vi "UHR-Fleezers Control (host) - 10.8MV_trial.vi"() -> ()   [LabVIEW 2010] (continued)
    n1525 = Multiply(x=10.0, y=w5371) -> (x*y=→"Trap 1 Position RMS (A)":dbl)
    n1526 = Divide(x=w5471, y=w5467) -> (x/y=w5439:waveform(dbl)[])
    n1527 = Index Array(array=w5439, index=0) -> (element=w5449:waveform(dbl))
    n1528 = case "For computing FFTs for display" shown="True" "Compute FFT" {
      tunnel: w5466 -> [_ w7792]
      frame False {
      }
      frame True {
        n1529 = Build Array("FFT 1 Choice 1", "FFT 1 Choice 2", "FFT 2 Choice 1", "FFT 2 Choice 2") -> (w7785:u16[])
        n1530 = Array Size(array=w7792) -> (size(s)=w7791:i32)
        n1531 = feedback-in #6(w7785) -> ()
        n1532 = feedback #6(u16[] [100, 100, 100, 100]) -> (w7786:u16[])
        n1533 = feedback-in #7("# Spectra to Ave.") -> ()
        n1534 = feedback #7("# Spectra to Ave.") -> (w7783:dbl)
        n1535 = Not Equal?(x="# Spectra to Ave.", y=w7783) -> (x != y?=w7782:bool)
        n1536 = Not Equal?(x=w7785, y=w7786) -> (x != y?=w7784:bool)
        n1537 = feedback #8(1.0) -> (w7769:dbl)
        n1538 = Compound Arithmetic op=OR("Reset FFT", w7784, w7782) -> (w7767:bool)
        n1539 = Select(t=1.0, s=w7767, f=w7769) -> (s? t:f=w7771:dbl)
        n1540 = Greater?(x=w7771, y="# Spectra to Ave.") -> (0:w7790:bool)
        n1541 = Increment(x=w7771) -> (x+1=w7770:dbl)
        n1542 = feedback-in #8(w7770) -> ()
        n1543 = local read "DMA Update Period (s)"() -> (w7765:dbl)
        n1544 = Multiply(x="# Spectra to Ave.", y=w7765) -> (x*y=→"Ave. Time (s)":dbl)
        n1545 = Build Array(cluster{"f0":dbl, "df":dbl, "magnitude":dbl[]} {"f0"=0.0, "df"=0.0, "magnitude"=[]} ("PSD")) -> (w7774:cluster{"f0":dbl, "df":dbl, "magnitude":dbl[]}[])
        n1546 = Build Array(w7774, w7774, w7774, w7774) -> (w7776:T49)
        n1547 = feedback #9(w7776) -> (w7781:T49)
        n1548 = for {
          N: 4 -> [_]
          tunnel: w7785 -> [w7814] mode=indexing
          tunnel: w7792 -> [w7815]
          tunnel: w7791 -> [w7817]
          tunnel: w7767 -> [w7810]
          tunnel: w7790 -> [w7809]
          tunnel: "# Spectra to Ave." -> [w7808]
          tunnel: [w7807] -> w7780 mode=indexing
          tunnel: w7781 -> [w7812] mode=indexing
          tunnel: [w7811] -> w7768 mode=indexing
          tunnel: w7771 -> [w7806]
          n1549 = Less?(x=w7814, y=w7817) -> (x < y?=w7816:bool)
          n1550 = Index Array(array=w7815, index=w7814) -> (element=w7813:waveform(dbl))
          n1551 = case shown="True" w7816 {
            tunnel: w7813 -> [_ w7834]
            tunnel: w7812 -> [w7819 w7832]
            tunnel: [w7819 w7820] -> w7811
            tunnel: w7810 -> [_ w7831]
            tunnel: w7809 -> [_ w7824]
            tunnel: w7808 -> [_ w7823]
            tunnel: [cluster{"f0":dbl, "df":dbl, "magnitude":dbl[]} {"f0"=0.0, "df"=0.0, "magnitude"=[]} ("PSD") w7825] -> w7807
            tunnel: w7806 -> [_ w7822]
            frame False {
            }
            frame True {
              n1552 = call <vilib>:"Std Deviation and Variance.vi"("X"=w7834) -> ("mean"=w7835:dbl)  [unwired: 1 in, 2 out]
              n1553 = Subtract(x=w7834, y=w7835) -> (x-y=w7833:waveform(dbl))
              n1554 = xnode "Spectral Measurements"("Signals"=w7833) -> ("PSD"=w7827:cluster{"f0":dbl, "df":dbl, "magnitude":dbl[]})  [unwired: 1 in, 1 out]
              n1555 = case shown="False" w7831 {
                tunnel: w7832 -> [w7844 _]
                tunnel: [w7840 w7849] -> w7820
                tunnel: w7827 -> [w7843 w7850]
                tunnel: w7824 -> [w7842 _]
                frame False {
                  n1556 = Build Array (concatenate)(w7844, w7843) -> (w7841:cluster{"f0":dbl, "df":dbl, "magnitude":dbl[]}[])
                  n1557 = case shown="True" w7842 {
                    tunnel: w7841 -> [w7845 w7848]
                    tunnel: [w7845 w7846] -> w7840
                    frame False {
                    }
                    frame True {
                      n1558 = Delete From Array(array=w7848, index=0) -> (array with subset deleted=w7846:cluster{"f0":dbl, "df":dbl, "magnitude":dbl[]}[])  [unwired: 1 in, 1 out]
                    }
                  }
                }
                frame True {
                  n1559 = Build Array(w7850) -> (w7849:cluster{"f0":dbl, "df":dbl, "magnitude":dbl[]}[])
                }
              }
              n1560 = for {
                tunnel: w7820 -> [w7839] mode=indexing
                tunnel: [w7838] -> w7830 mode=indexing
                workers-P: _ -> [_]
                n1561 = Unbundle By Name(w7839) -> ("magnitude"=w7838:dbl[])
              }
              n1562 = Transpose 2D Array(2D array=w7830) -> (transposed array=w7829:dbl[][])
              n1563 = for {
                tunnel: w7829 -> [w7837] mode=indexing
                tunnel: [w7836] -> w7828 mode=indexing
                workers-P: _ -> [_]
                n1564 = Add Array Elements(numeric array=w7837) -> (sum=w7836:dbl)
              }
              n1565 = Select(t=w7823, s=w7824, f=w7822) -> (s? t:f=w7821:dbl)
              n1566 = Divide(x=w7828, y=w7821) -> (x/y=w7826:dbl[])
              n1567 = Bundle By Name(cluster=w7827, "magnitude"=w7826) -> (w7825:cluster{"f0":dbl, "df":dbl, "magnitude":dbl[]})
            }
          }
        }
        n1568 = case shown="True" w7767 {
          tunnel: w7768 -> [w7799 w7805]
          tunnel: [w7799 w7800] -> w7766
          frame False {
          }
          frame True {
            n1569 = Array Subset(array=w7805, index (row)=0 ("index"), length (row)=4 ("length"), index (col)=0 ("index"), length (col)=1 ("length")) -> (w7800:T49)
          }
        }
        n1570 = feedback-in #9(w7766) -> ()
        n1571 = Split 1D Array(array=w7780, index=2) -> (first subarray=→"FFT 1":cluster{"f0":dbl, "df":dbl, "magnitude":dbl[]}[], second subarray=→"FFT 2":cluster{"f0":dbl, "df":dbl, "magnitude":dbl[]}[])
      }
    }
    n1572 = Index Array(array=w5439, index=1) -> (element=w5447:waveform(dbl))
    n1573 = case "For displaying the high resolution display (no downsampling)" shown="True" w5512 {
      tunnel: w5466 -> [_ w5974]
      frame False {
      }
      frame True {
        n1574 = Index Array(array=w5974, index="High Res. Display") -> (element=w5975:waveform(dbl))
        n1575 = call <vilib>:"Std Deviation and Variance.vi"("X"=w5975) -> ("mean"=w5982:dbl, "standard deviation"=w5987:dbl)  [unwired: 1 in, 1 out]
        "Mean Intensity" <- w5982
        "Sigma" <- w5987
        n1576 = Subtract(x=w5975, y=w5982) -> (x-y=w5981:waveform(dbl))
        n1577 = Select(t=w5981, s="Subtract mean", f=w5975) -> (s? t:f=→"1 Channel":waveform(dbl))
        n1578 = Divide(x=w5987, y=w5982) -> (x/y=→"Sigma/Mean":dbl)
        n1579 = feedback #10(1) -> (w5976:i32)
        n1580 = Greater Or Equal?(x=w5976, y="Slow mean N ave.") -> (x >= y?=w5989:bool)
        n1581 = Increment(x=w5976) -> (x+1=w5991:i32)
        n1582 = Select(t=1, s=w5989, f=w5991) -> (s? t:f=w5978:i32)
        n1583 = feedback-in #10(w5978) -> ()
        n1584 = feedback #11() -> (w5979:waveform(dbl))  [unwired: 1 out]
        n1585 = case shown="Default" w5976 {
          tunnel: [w5994 w5997] -> w5980
          tunnel: w5979 -> [w5996 _]
          tunnel: w5975 -> [w5995 w5997]
          frame Default {
            n1586 = call-poly <vilib>:"Append Waveforms.vi"("waveform B"=w5995, "waveform A"=w5996) -> ("waveform out"=w5994:waveform(dbl))  [unwired: 1 in, 8 out]
          }
          frame 1 {
          }
        }
        n1587 = feedback-in #11(w5980) -> ()
        n1588 = case shown="True" w5989 {
          tunnel: w5980 -> [_ w5993]
          frame False {
          }
          frame True {
            n1589 = call <vilib>:"Mean.vi"("X"=w5993) -> ("mean"=→"Slow mean":dbl)  [unwired: 1 out]
          }
        }
      }
    }
    n1590 = case "For plotting results of scanning MCL" shown="True" w5589 {
      tunnel: w5588 -> [_ w6505]
      tunnel: w5505 -> [_ w6601]
      tunnel: w5597 -> [_ _]
      tunnel: w5466 -> [_ w6575]
      tunnel: w5441 -> [_ w6506]
      tunnel: w5440 -> [_ w6479]
      frame False {
      }
      frame True {
        w6486 = u32 0 items=["Horizontal", "Vertical", "Central", "1st Diagonal", "2nd Diagonal"] ("Type of Symmetry")
        w6514 = u32 0 items=["Horizontal", "Vertical", "Central", "1st Diagonal", "2nd Diagonal"] ("Type of Symmetry")
        w6517 = u32 0 items=["Horizontal", "Vertical", "Central", "1st Diagonal", "2nd Diagonal"] ("Type of Symmetry")
        w6546 = u32 0 items=["Horizontal", "Vertical", "Central", "1st Diagonal", "2nd Diagonal"] ("Type of Symmetry")
        n1591 = Index Array(array=w6575, index=10) -> (element=w6581:waveform(dbl))
        n1592 = Index Array(array=w6575, index=11) -> (element=w6578:waveform(dbl))
        n1593 = local read "Cycles/step (MCL)"() -> (w6531:u64)
        n1594 = Index Array(array=w6575, index="Channel") -> (element=w6577:waveform(dbl))
        n1595 = Unbundle(w6479) -> ("New Image"=w6478:T2, "New Image"=w6477:T2, "New Image"=w6476:T2, "New Image"=w6475:T2)
        n1596 = Unbundle By Name(w6581) -> ("Y"=w6533:dbl[])
        n1597 = Unbundle By Name(w6578) -> ("Y"=w6535:dbl[])
        n1598 = Unbundle By Name(w6577) -> ("Y"=w6540:dbl[])
        n1599 = call "downsample 1D array - double.vi"("Ave N"=w6531, "Array In"=w6533) -> ("Array Out"=w6532:dbl[])  [unwired: 1 out]
        n1600 = call "downsample 1D array - double.vi"("Ave N"=w6531, "Array In"=w6535) -> ("Array Out"=w6534:dbl[])  [unwired: 1 out]
        n1601 = call "downsample 1D array - double.vi"("Ave N"=w6531, "Array In"=w6540) -> ("Array Out"=w6539:dbl[])  [unwired: 1 out]
        n1602 = feedback #12(w6601) -> (w6602:dbl[])
        n1603 = Build Array (concatenate)(w6602, w6601) -> (w6583:dbl[])
        n1604 = feedback #13(w6506) -> (w6508:dbl[])
        n1605 = Build Array (concatenate)(w6508, w6506) -> (w6507:dbl[])
        n1606 = local read "Scan steps (MCL)"() -> (w6488:u64)
        n1607 = Select(t=w6601, s=w6505, f=w6583) -> (s? t:f=w6587:dbl[])
        n1608 = feedback-in #12(w6587) -> ()
        n1609 = Select(t=w6506, s=w6505, f=w6507) -> (s? t:f=w6489:dbl[])
        n1610 = feedback-in #13(w6489) -> ()
        n1611 = local read "Scan lines (y)"() -> (w6474:u64)
        n1612 = local read "N APD Samp/step"() -> (w6490:dbl)
        n1613 = feedback #14(w6532) -> (w6589:dbl[])
        n1614 = Build Array (concatenate)(w6589, w6532) -> (w6580:dbl[])
        n1615 = feedback #15(w6539) -> (w6599:dbl[])
        n1616 = Build Array (concatenate)(w6599, w6539) -> (w6598:dbl[])
        n1617 = feedback #16(w6534) -> (w6591:dbl[])
        n1618 = Build Array (concatenate)(w6591, w6534) -> (w6592:dbl[])
        n1619 = Select(t=w6532, s=w6505, f=w6580) -> (s? t:f=w6536:dbl[])
        n1620 = feedback-in #14(w6536) -> ()
        n1621 = Select(t=w6539, s=w6505, f=w6598) -> (s? t:f=w6538:dbl[])
        n1622 = feedback-in #15(w6538) -> ()
        n1623 = Select(t=w6534, s=w6505, f=w6592) -> (s? t:f=w6537:dbl[])
        n1624 = feedback-in #16(w6537) -> ()
        n1625 = Multiply(x=w6488, y=u64 2) -> (x*y=w6473:u64)
        n1626 = call "integrate 1D array interval - double.vi"("Ave N"=w6490, "Array In"=w6489) -> ("Array Out"=w6501:dbl[])  [unwired: 1 out]
        n1627 = call "integrate 1D array interval - double.vi"("Ave N"=w6490, "Array In"=w6587) -> ("Array Out"=w6586:dbl[])  [unwired: 1 out]
        n1628 = Array Size(array=w6501) -> (size(s)=w6502:i32)
        n1629 = Array Size(array=w6586) -> (size(s)=w6588:i32)
        n1630 = Multiply(x=w6474, y=w6473) -> (x*y=w6504:u64)
        n1631 = Multiply(x=w6474, y=w6473) -> (x*y=w6596:u64)
        n1632 = call <vilib>:"Mean.vi"("X"=w6536) -> ("mean"=w6520:dbl)  [unwired: 1 out]
        n1633 = Subtract(x=w6504, y=w6502) -> (x-y=w6495:u64)
        n1634 = call <vilib>:"Mean.vi"("X"=w6538) -> ("mean"=w6525:dbl)  [unwired: 1 out]
        n1635 = call <vilib>:"Mean.vi"("X"=w6537) -> ("mean"=w6523:dbl)  [unwired: 1 out]
        n1636 = call <vilib>:"Mean.vi"("X"=w6501) -> ("mean"=w6492:dbl)  [unwired: 1 out]
        n1637 = Subtract(x=w6596, y=w6588) -> (x-y=w6530:u64)
        n1638 = call <vilib>:"Mean.vi"("X"=w6586) -> ("mean"=w6527:dbl)  [unwired: 1 out]
        n1639 = Initialize Array(1.0 ("element"), w6495) -> (w6491:dbl[])
        n1640 = Initialize Array(1.0 ("element"), w6530) -> (w6521:dbl[])
        n1641 = Multiply(x=w6491, y=w6492) -> (x*y=w6493:dbl[])
        n1642 = Multiply(x=w6521, y=w6523) -> (x*y=w6524:dbl[])
        n1643 = Multiply(x=w6521, y=w6525) -> (x*y=w6526:dbl[])
        n1644 = Multiply(x=w6521, y=w6520) -> (x*y=w6522:dbl[])
        n1645 = Multiply(x=w6521, y=w6527) -> (x*y=w6528:dbl[])
        n1646 = Build Array (concatenate)(w6536, w6522) -> (w6590:dbl[])
        n1647 = Build Array (concatenate)(w6538, w6526) -> (w6594:dbl[])
        n1648 = Build Array (concatenate)(w6537, w6524) -> (w6593:dbl[])
        n1649 = Build Array (concatenate)(w6501, w6493) -> (w6503:dbl[])
        n1650 = Build Array (concatenate)(w6586, w6528) -> (w6595:dbl[])
        n1651 = Reshape Array(w6590, w6474, w6473) -> (w6556:dbl[][])
        n1652 = Reshape Array(w6503, w6474, w6473) -> (w6499:dbl[][])
        n1653 = Reshape Array(w6594, w6474, w6473) -> (w6548:dbl[][])
        n1654 = Reshape Array(w6593, w6474, w6473) -> (w6563:dbl[][])
        n1655 = Reshape Array(w6595, w6474, w6473) -> (w6573:dbl[][])
        n1656 = Array Subset(array=w6563, index (col)=0 ("index"), length (col)=w6488) -> (w6568:dbl[][])  [unwired: 2 in]
        n1657 = Array Subset(array=w6563, index (col)=w6488) -> (w6566:dbl[][])  [unwired: 3 in]
        n1658 = Array Subset(array=w6548, index (col)=0 ("index"), length (col)=w6488) -> (w6554:dbl[][])  [unwired: 2 in]
        n1659 = Array Subset(array=w6548, index (col)=w6488) -> (w6552:dbl[][])  [unwired: 3 in]
        n1660 = Array Subset(array=w6499, index (col)=0 ("index"), length (col)=w6488) -> (w6498:dbl[][])  [unwired: 2 in]
        n1661 = Array Subset(array=w6499, index (col)=w6488) -> (w6496:dbl[][])  [unwired: 3 in]
        n1662 = Array Subset(array=w6573, index (col)=0 ("index"), length (col)=w6488) -> (w6572:dbl[][])  [unwired: 2 in]
        n1663 = Array Subset(array=w6573, index (col)=w6488) -> (w6570:dbl[][])  [unwired: 3 in]
        n1664 = Array Subset(array=w6556, index (col)=0 ("index"), length (col)=w6488) -> (w6561:dbl[][])  [unwired: 2 in]
        n1665 = Array Subset(array=w6556, index (col)=w6488) -> (w6559:dbl[][])  [unwired: 3 in]
        n1666 = for {
          tunnel: w6568 -> [w6610] mode=indexing
          tunnel: [w6609] -> w6567 mode=indexing
          workers-P: _ -> [_]
          n1667 = Reverse 1D Array(array=w6610) -> (reversed array=w6609:dbl[])
        }
        n1668 = for {
          tunnel: w6554 -> [w6606] mode=indexing
          tunnel: [w6605] -> w6553 mode=indexing
          workers-P: _ -> [_]
          n1669 = Reverse 1D Array(array=w6606) -> (reversed array=w6605:dbl[])
        }
        n1670 = for {
          tunnel: w6498 -> [w6604] mode=indexing
          tunnel: [w6603] -> w6497 mode=indexing
          workers-P: _ -> [_]
          n1671 = Reverse 1D Array(array=w6604) -> (reversed array=w6603:dbl[])
        }
        n1672 = for {
          tunnel: w6572 -> [w6612] mode=indexing
          tunnel: [w6611] -> w6571 mode=indexing
          workers-P: _ -> [_]
          n1673 = Reverse 1D Array(array=w6612) -> (reversed array=w6611:dbl[])
        }
        n1674 = for {
          tunnel: w6561 -> [w6608] mode=indexing
          tunnel: [w6607] -> w6560 mode=indexing
          workers-P: _ -> [_]
          n1675 = Reverse 1D Array(array=w6608) -> (reversed array=w6607:dbl[])
        }
        n1676 = Index Array(array=w6573, index (row)=0) -> (element=→"Waveform Graph":dbl[])  [unwired: 1 in]
        n1677 = Add(x=w6567, y=w6566) -> (x+y=w6565:dbl[][])
        n1678 = Add(x=w6553, y=w6552) -> (x+y=w6551:dbl[][])
        n1679 = Add(x=w6497, y=w6496) -> (x+y=w6481:dbl[][])
        n1680 = Add(x=w6571, y=w6570) -> (x+y=w6545:dbl[][])
        n1681 = Add(x=w6560, y=w6559) -> (x+y=w6558:dbl[][])
        n1682 = Divide(x=w6551, y=2) -> (x/y=w6549:dbl[][])
        n1683 = Divide(x=w6565, y=2) -> (x/y=w6510:dbl[][])
        n1684 = Divide(x=w6558, y=2) -> (x/y=w6512:dbl[][])
        n1685 = To Single Precision Float(number=w6545) -> (single precision float=w6544:sgl[][])
        n1686 = Transpose 2D Array(2D array=w6549) -> (transposed array=→"Data map":dbl[][])
        n1687 = To Single Precision Float(number=w6481) -> (single precision float=w6485:sgl[][])
        n1688 = To Single Precision Float(number=w6510) -> (single precision float=w6516:sgl[][])
        n1689 = To Single Precision Float(number=w6512) -> (single precision float=w6513:sgl[][])
        n1690 = call "IMAQ ArrayToImage"("Image Pixels (Float)"=w6544, "Image"=w6478) -> ("Image Out"=w6547:T2)  [unwired: 8 in, 1 out]
        n1691 = call "IMAQ ArrayToImage"("Image Pixels (Float)"=w6485, "Image"=w6477) -> ("Image Out"=w6487:T2)  [unwired: 8 in, 1 out]
        n1692 = call "IMAQ ArrayToImage"("Image Pixels (Float)"=w6516, "Image"=w6476) -> ("Image Out"=w6518:T2)  [unwired: 8 in, 1 out]
        n1693 = call "IMAQ ArrayToImage"("Image Pixels (Float)"=w6513, "Image"=w6475) -> ("Image Out"=w6515:T2)  [unwired: 8 in, 1 out]
        n1694 = call "IMAQ Symmetry"("Type of Symmetry"=w6546, "Image Src"=w6547) -> ("Image Dst Out"=w6542:T2)  [unwired: 3 in, 1 out]
        n1695 = call "IMAQ Symmetry"("Type of Symmetry"=w6486, "Image Src"=w6487) -> ("Image Dst Out"=w6483:T2)  [unwired: 3 in, 1 out]
        n1696 = call "IMAQ Symmetry"("Type of Symmetry"=w6517, "Image Src"=w6518) -> ("Image Dst Out"=→"Detection Laser X":T2)  [unwired: 3 in, 1 out]
        n1697 = call "IMAQ Symmetry"("Type of Symmetry"=w6514, "Image Src"=w6515) -> ("Image Dst Out"=→"Detection Laser Y":T2)  [unwired: 3 in, 1 out]
        n1698 = call "IMAQ Set Simple Calibration"("Calibration Axis Info"=T38 {"Origin Pixel"={"X"=0.0, "Y"=0.0}, "Angle Relative to Horizontal (deg)"=0.0, "Axis Reference"=0}, "Grid Descriptor"=T39 {"X Step"=0.3, "Y Step"=0.3, "Unit"=enum."Undefined"}, "Image"=w6542) -> ("Calibrated Image"=→"APD 1":T2)  [unwired: 7 in, 1 out]
        n1699 = call "IMAQ Set Simple Calibration"("Calibration Axis Info"=T38 {"Origin Pixel"={"X"=0.0, "Y"=0.0}, "Angle Relative to Horizontal (deg)"=0.0, "Axis Reference"=0}, "Grid Descriptor"=T39 {"X Step"=0.3, "Y Step"=0.3, "Unit"=enum."Undefined"}, "Image"=w6483) -> ("Calibrated Image"=→"APD 2":T2)  [unwired: 7 in, 1 out]
      }
    }
    n1700 = Subtract(x=w5447, y="APD 2 Offset") -> (x-y=w5444:waveform(dbl))
    n1701 = Subtract(x=w5449, y="APD 1 Offset") -> (x-y=w5445:waveform(dbl))
    n1702 = Index Array(array=w5464, index=3) -> (element=w5533:waveform(dbl))
    n1703 = Index Array(array=w5464, index=6) -> (element=w5530:waveform(dbl))
    n1704 = Build Array(w5445, w5444) -> (→"APD Chart":waveform(dbl)[])
    n1705 = Array Size(array=w5522) -> (size(s)=w5577:i32)
    n1706 = call <vilib>:"Std Deviation and Variance.vi"("X"=w5457) -> ("standard deviation"=w5456:dbl)  [unwired: 1 in, 2 out]
    n1707 = Add Array Elements(numeric array=w5457) -> (sum=w5459:u32)
    n1708 = Add Array Elements(numeric array=w5522) -> (sum=w5587:u32)
    n1709 = call <vilib>:"Std Deviation and Variance.vi"("X"=w5522) -> ("standard deviation"=w5521:dbl)  [unwired: 1 in, 2 out]
    n1710 = Divide(x="T1 offset_x (mV)", y=1000.0) -> (x/y=w5534:dbl)
    n1711 = Divide(x=w5456, y=w5455) -> (x/y=w5452:dbl)
    "Rate sigma (Hz) 2" <- w5452
    n1712 = Multiply(x=w5455, y=w5577) -> (x*y=w5458:dbl)
    "Int. Time (s)" <- w5458
    n1713 = Divide(x=w5459, y=w5458) -> (x/y=w5453:dbl)
    "APD 2 Rate (Hz)" <- w5453
    n1714 = Divide(x=w5587, y=w5458) -> (x/y=w5519:dbl)
    "APD 1 Rate (Hz)" <- w5519
    n1715 = Divide(x=w5521, y=w5455) -> (x/y=w5520:dbl)
    "Rate sigma (Hz)" <- w5520
    n1716 = Divide(x=w5452, y=w5453) -> (x/y=→"Sigma/Mean 2":dbl)
    n1717 = Divide(x=w5520, y=w5519) -> (x/y=→"Sigma/Mean":dbl)
    n1718 = Divide(x="T2 offset_x (mV)", y=1000.0) -> (x/y=w5532:dbl)
    n1719 = case shown="1" "Calibration" {
      tunnel: "T1 alpha_x (nm/V)" -> [_ w6441 w6462]
      tunnel: "T1 kappa_x (pN/nm)" -> [_ _ w6452]
      tunnel: "T2 alpha_x (nm/V)" -> [_ w6440 w6460]
      tunnel: "T2 kappa_x (pN/nm)" -> [_ _ w6453]
      tunnel: w5533 -> [w6423 w6438 w6458]
      tunnel: w5530 -> [w6422 w6436 w6456]
      tunnel: [w6423 w6435 w6455] -> w5563
      tunnel: [w6422 w6434 w6454] -> w5562
      tunnel: ["T1 X (V)" ("Label.Text") "T1 X (nm)" ("Label.Text") "T1 X (pN)" ("Label.Text")] -> w5551
      tunnel: ["T2 X (V)" ("Label.Text") "T2 X (nm)" ("Label.Text") "T2 X (pN)" ("Label.Text")] -> w5550
      tunnel: ["Position (V)" ("Label.Text") "Position (nm)" ("Label.Text") "Force (pN)" ("Label.Text")] -> w5552
      tunnel: w5532 -> [_ w6426 w6445]
      tunnel: w5534 -> [_ w6429 w6447]
      tunnel: ["Mean (V)" ("Label.Text") "Mean (nm)" ("Label.Text") "Mean (pN)" ("Label.Text")] -> w5547
      tunnel: ["Difference (V)" ("Label.Text") "Difference (nm)" ("Label.Text") "Difference (pN)" ("Label.Text")] -> w5472
      frame 0, Default {
      }
      frame 1 {
        # "position"
        n1720 = Unbundle By Name(w6438) -> ("Y"=w6442:dbl[])
        n1721 = Unbundle By Name(w6436) -> ("Y"=w6427:dbl[])
        n1722 = Subtract(x=w6442, y=w6429) -> (x-y=w6430:dbl[])
        n1723 = Subtract(x=w6427, y=w6426) -> (x-y=w6428:dbl[])
        n1724 = Multiply(x=w6428, y=w6440) -> (x*y=w6437:dbl[])
        n1725 = Multiply(x=w6441, y=w6430) -> (x*y=w6439:dbl[])
        n1726 = Bundle By Name(cluster=w6436, "Y"=w6437) -> (w6434:waveform(dbl))
        n1727 = Bundle By Name(cluster=w6438, "Y"=w6439) -> (w6435:waveform(dbl))
      }
      frame 2 {
        # "force"
        n1728 = Unbundle By Name(w6458) -> ("Y"=w6463:dbl[])
        n1729 = Unbundle By Name(w6456) -> ("Y"=w6461:dbl[])
        n1730 = Subtract(x=w6461, y=w6445) -> (x-y=w6446:dbl[])
        n1731 = Subtract(x=w6463, y=w6447) -> (x-y=w6448:dbl[])
        n1732 = Compound Arithmetic op=MULTIPLY(w6446, w6460, w6453) -> (w6457:dbl[])
        n1733 = Compound Arithmetic op=MULTIPLY(w6452, w6462, w6448) -> (w6459:dbl[])
        n1734 = Bundle By Name(cluster=w6456, "Y"=w6457) -> (w6454:waveform(dbl))
        n1735 = Bundle By Name(cluster=w6458, "Y"=w6459) -> (w6455:waveform(dbl))
      }
    }
    n1736 = feedback-in #17("Calibration") -> ()
    n1737 = feedback #17(u16 1 ("Calibration")) -> (w5554:u16)
    n1738 = Not Equal?(x=w5554, y="Calibration") -> (x != y?=w5510:bool)
    n1739 = Unbundle By Name(w5533) -> ("Y"=w5536:dbl[])
    n1740 = Unbundle By Name(w5530) -> ("Y"=w5539:dbl[])
    n1741 = Subtract(x=w5536, y=w5534) -> (x-y=w5537:dbl[])
    n1742 = Subtract(x=w5539, y=w5532) -> (x-y=w5538:dbl[])
    n1743 = disable-structure shown="Enabled" {
      disable-tunnel: [-1.0 ("y") 1.0] -> w5540
      frame Disabled {
      }
      frame Enabled {
      }
    }
    n1744 = Multiply(x=w5538, y="T2 alpha_x (nm/V)") -> (x*y=w5529:dbl[])
    n1745 = Multiply(x="T1 alpha_x (nm/V)", y=w5537) -> (x*y=w5528:dbl[])
    n1746 = Multiply(x=w5562, y=w5540) -> (x*y=w5541:waveform(dbl))
    n1747 = case shown="True" "Read Lateness and Rel Phase" {
      tunnel: w5364 -> [w5998 w6020]
      tunnel: w5363 -> [w5999 w6019]
      tunnel: [w5998 w6018] -> w5525
      tunnel: [w5999 w6017] -> w5524
      frame False {
      }
      frame True {
        n1748 = xnode "Read/Write Control"("FPGA VI Reference In"=w6020, "error in"=w6019) -> ("FPGA VI Reference Out"=w6018:T19, "error out"=w6017:errorcluster, "GI Relative phase"=→"GI relative phase":i16, "Relative phase"=→"Relative phase (AI1)":i16, "AI Late Counter"=→"Late Counter (AI1)":u16, "GI Late Counter"=→"GI Late Counter":u16, "MCL Late Counter"=→"MCL Late Counter":u16, "MCL Relative Phase"=→"Relative Phase (MCL)":i16, "APD Acq Relative Phase"=→"APD Acq Relative Phase":i16, "APD 1 Gate Relative Phase"=→"APD 1 Gate Relative Phase":i16, "APD 2 Gate Relative Phase"=→"APD 2 Gate Relative Phase":i16, "APD Acq Late Counter"=→"APD Acq Late Counter":u16, "APD 1 Gate Late Counter"=→"APD 1 Gate Late Counter":u16, "APD 2 Gate Late Counter"=→"APD 2 Gate Late Counter":u16, "Green FB Relative Phase"=→"Relative phase (Green FB)":i16, "GI Relative phase 2"=→"GI relative phase 2":i16, "GI Late Counter 2"=→"GI Late Counter 2":u16, "Trap Pos FIFO Timeout"=→"Trap Pos FIFO Timeout":u16, "Trap AI FIFO Timeout"=→"Trap AI FIFO Timeout":u16)
      }
    }
    n1749 = Subtract(x=w5529, y=w5528) -> (x-y=w5527:dbl[])
    n1750 = Unbundle By Name(w5562) -> ("Y"=w5497:dbl[])
    n1751 = Unbundle By Name(w5563) -> ("Y"=w5498:dbl[])
    n1752 = Build Array(w5563, w5541) -> (→"Force":waveform(dbl)[])
    n1753 = Subtract(x=w5527, y="Offset (nm)") -> (x-y=w5495:dbl[])
    n1754 = call <vilib>:"Mean.vi"("X"=w5497) -> ("mean"=w5476:dbl)  [unwired: 1 out]
    "T2 X" <- w5476
    n1755 = Absolute Value(x=w5498) -> (abs(x)=w5499:dbl[])
    n1756 = Absolute Value(x=w5497) -> (abs(x)=w5500:dbl[])
    n1757 = call <vilib>:"Mean.vi"("X"=w5498) -> ("mean"=w5477:dbl)  [unwired: 1 out]
    "T1 X" <- w5477
    n1758 = Add(x=w5499, y=w5500) -> (x+y=w5501:dbl[])
    n1759 = Bundle By Name(cluster=w5533, "Y"=w5495) -> (w5463:waveform(dbl))
    "Bead Separation" <- w5463
    n1760 = Divide(x=w5501, y=2.0) -> (x/y=→"Vec Mean of T1 T2":dbl[])
    n1761 = case shown="True" w5510 {
      tunnel: w5552 -> [_ w6416]
      tunnel: w5551 -> [_ w6415]
      tunnel: w5550 -> [_ w6414]
      tunnel: w5547 -> [_ w6413]
      tunnel: w5472 -> [_ w6412]
      frame False {
      }
      frame True {
        n1762 = property on="Force" class="WFChart (strict)"("YScale.NameLbl.Text"=w6416) -> ()  [unwired: 2 in, 2 out]
        n1763 = property on="T2 X" class="DigNum (strict)"("Caption.Text"=w6414) -> ()  [unwired: 2 in, 2 out]
        n1764 = property on="T1 X" class="DigNum (strict)"("Caption.Text"=w6415) -> ()  [unwired: 2 in, 2 out]
        n1765 = property on="Mean" class="DigNum (strict)"("Caption.Text"=w6413) -> ()  [unwired: 2 in, 2 out]
        n1766 = property on="Difference" class="DigNum (strict)"("Caption.Text"=w6412) -> ()  [unwired: 2 in, 2 out]
      }
    }
    n1767 = local read "Tether"() -> (w5504:bool)
    n1768 = Absolute Value(x=w5477) -> (abs(x)=w5474:dbl)
    n1769 = Absolute Value(x=w5476) -> (abs(x)=w5473:dbl)
    n1770 = Add(x=w5474, y=w5473) -> (x+y=w5549:dbl)
    n1771 = Subtract(x=w5474, y=w5473) -> (x-y=→"Difference":dbl)
    n1772 = feedback #18(w5495) -> (w5494:dbl[])
    n1773 = Divide(x=w5549, y=2.0) -> (x/y=w5503:dbl)
    "Mean" <- w5503
    n1774 = case shown="True" w5504 {
      tunnel: w5503 -> [_ w5957]
      frame False {
      }
      frame True {
        n1775 = Greater?(x="Lost Tether Alarm Threshold (pN)", y=w5957) -> (0:w5955:bool)
        n1776 = case shown="True" w5955 {
          frame False {
          }
          frame True {
            n1777 = flat-sequence {
              frame #0 {
                # "stop only if saving"
                n1778 = local read "Saving..."() -> (w5970:bool)
                n1779 = And(x=w5970, y="TA Cancel Save?") -> (x .and. y?=w5969:bool)
                n1780 = local write "Stop Saving"(w5969) -> ()
              }
              frame #1 {
                n1781 = case shown="True" "TA Green Off?" {
                  frame False {
                  }
                  frame True {
                    w5973 = FALSE ("Fl. Triggered...")
                    n1782 = local write "Fl. Triggered..."(w5973) -> ()
                    n1783 = property on="Green Laser ON/Interlacing" class="Bool (strict)"("Val(Sgnl)"=w5973) -> ()  [unwired: 2 in, 2 out]
                  }
                }
              }
            }
            n1784 = local read "Time tether formed"() -> (w5964:timestamp)
            n1785 = Get Date/Time In Seconds() -> (seconds since 1Jan1904=w5965:timestamp)
            n1786 = Subtract(x=w5965, y=w5964) -> (x-y=w5963:dbl)
            n1787 = Number To Decimal String(number=w5963) -> (decimal integer string=w5960:string)  [unwired: 1 out]
            n1788 = local read "Messages"() -> (w5967:string)
            n1789 = call <vilib>:"Beep.vi"() -> ()  [unwired: 3 in, 9 out]
            n1790 = Concatenate Strings("Lost tether (" ("Message to add"), w5960, " s)." ("string")) -> (w5962:string)
            n1791 = local write "Tether"(FALSE ("Tether")) -> ()
            n1792 = call "Update messages.vi"("Message to add"=w5962, "Old message string"=w5967) -> ("New message string"=w5966:string)
            n1793 = local write "Messages"(w5966) -> ()
            n1794 = property on="Trap Pos. FB ON" class="Bool (strict)"("Val(Sgnl)"=FALSE ("Value (Signaling)")) -> ()  [unwired: 2 in, 2 out]
          }
        }
      }
    }
    n1795 = Build Array (concatenate)(w5495, w5494) -> (w5493:dbl[])
    n1796 = Split 1D Array(array=w5493, index=w5375) -> (first subarray=w5489:dbl[])  [unwired: 1 out]
    n1797 = feedback-in #18(w5489) -> ()
    n1798 = call <vilib>:"Mean.vi"("X"=w5489) -> ("mean"=w5488:dbl)  [unwired: 1 out]
    "Bead Mean (nm)" <- w5488
    n1799 = Subtract(x=w5489, y=w5488) -> (x-y=w5487:dbl[])
    n1800 = Square(x=w5487) -> (x^2=w5486:dbl[])
    n1801 = call <vilib>:"Mean.vi"("X"=w5486) -> ("mean"=w5485:dbl)  [unwired: 1 out]
    n1802 = Square Root(x=w5485) -> (sqrt(x)=w5484:dbl)
    n1803 = Multiply(x=10.0, y=w5484) -> (x*y=→"RMS (Ang)":dbl)
    n1804 = xnode "Read/Write Control"("FPGA VI Reference In"=w5525, "error in"=w5524) -> ("FPGA VI Reference Out"=w5643:T19, "error out"=w5637:errorcluster, "AI2 Y Sum Set 1"=w5633:i16, "AI2 Y Sum Set 2"=w5632:i16, "AI1 X Set 1"=w5409:fxp<+/-,16,1>, "AI1 X Set 2"=w5408:fxp<+/-,16,1>, "Trap Pos FB Int Signal"=→"Trap Pos FB Int Signal":fxp<+/-,24,9>, "Trap Pos FB Int-Norm Signal"=→"Trap Pos FB Int-Norm Signal":fxp<+/-,16,1>, "Trap Pos FB Action"=w5402:i64, "Scanning"=→"AOD Scanning":bool, "Scan I"=→"AOD Scan I":u64, "Scanning MCL"=w5635:bool, "Scan I (MCL)"=→"MCL Scan I":u64, "Green FB Signals"=w5572:T43)  [unwired: 1 out]
    "MCL Scanning" <- w5635
    "Trap Pos FB Action" <- w5402
    n1805 = local read "AI2 (V)"() -> (w5634:cluster{"Set 1":dbl, "Set 2":dbl})
    n1806 = Bundle By Name(cluster=w5634, "Set 1"=w5633, "Set 2"=w5632) -> (w5630:cluster{"Set 1":dbl, "Set 2":dbl})
    n1807 = Divide(x=w5402, y=327.67) -> (x/y=→"Action (%)":dbl)
    n1808 = local read "Trap X (AI1)"() -> (w5422:T10)
    n1809 = Divide(x=w5630, y=3276.7) -> (x/y=w5629:cluster{"Set 1":dbl, "Set 2":dbl})
    n1810 = local write "AI2 (V)"(w5629) -> ()
    n1811 = Bundle(cluster=w5422, "Trap 1"=w5409, "Trap 2"=w5408) -> (→"Trap X (AI1)":T10)
    n1812 = Divide(x=w5572, y=3276.7) -> (x/y=w5568:T50)
    n1813 = Unbundle By Name(w5568) -> ("Green FB Ch 0"=w5571:dbl, "Green FB Ch 1"=w5570:dbl, "Green FB Ch 2"=w5569:dbl)
    n1814 = Divide(x=w5571, y=w5569) -> (x/y=w5567:dbl)
    n1815 = Divide(x=w5570, y=w5569) -> (x/y=w5566:dbl)
    n1816 = flat-sequence "To save data" {
      tunnel: [w8273] -> w5654
      tunnel: [w8274] -> w5653
      tunnel: w5603 -> [w8267]
      tunnel: w5491 -> [w8271]
      tunnel: ["Save Calibration"] -> w5626
      tunnel: w5623 -> [w8270]
      tunnel: [w8263] -> w5622
      tunnel: [w8260] -> w5621
      tunnel: [w8257] -> w5620
      tunnel: w5602 -> [w8259]
      tunnel: w5508 -> [w8253]
      tunnel: [w8253] -> w5507
      tunnel: ["Start Saving"] -> w5465
      tunnel: [w8247] -> w5391
      tunnel: [w8246] -> w5390
      tunnel: w5654 -> [w8508]
      tunnel: w5653 -> [w8507]
      tunnel: w5392 -> [w8506]
      tunnel: w5626 -> [w8505]
      tunnel: w5622 -> [w8503]
      tunnel: w5621 -> [w8502]
      tunnel: w5620 -> [w8501]
      tunnel: w5478 -> [w8500]
      tunnel: w5517 -> [w8499]
      tunnel: w5507 -> [w8498]
      tunnel: w5465 -> [w8497]
      tunnel: w5463 -> [w8496]
      tunnel: w5439 -> [w8495]
      tunnel: w5391 -> [w8494]
      tunnel: w5390 -> [w8493]
      tunnel: w5389 -> [w8492]
      frame #0 {
        n1817 = Or(x="Save N Sets", y="Start Saving") -> (x .or. y?=w8254:bool)
        n1818 = To Double Precision Float(number=w8270) -> (double precision float=w8264:dbl)
        n1819 = Build Array(w8254, "Save Calibration", w8267, w8259) -> (w8269:bool[])
        n1820 = Compound Arithmetic op=OR("Save Calibration", w8267, w8254, w8259) -> (w8272:bool)
        n1821 = Boolean Array To Number(Boolean array=w8269) -> (number=w8266:u32)
        n1822 = feedback #19(FALSE ("Save APD Data\nwith Trap Data")) -> (w8248:bool)
        n1823 = feedback #20(refnum<k0> refnum) -> (w8275:refnum<file>)
        n1824 = feedback #21(refnum<k0> refnum) -> (w8250:refnum<file>)
        n1825 = feedback #22(FALSE ("Save APD Data\nwith Trap Data")) -> (w8258:bool)
        n1826 = feedback #23(refnum<k0> refnum) -> (w8261:refnum<file>)
        n1827 = feedback #24(0) -> (w8277:i32)
        n1828 = feedback #25() -> (w8265:u32)  [unwired: 1 out]
        n1829 = case shown="True" w8272 {
          tunnel: [w8284 1] -> w8273
          tunnel: w8277 -> [w8286 _]
          tunnel: [w8285 w8304] -> w8274
          tunnel: w8275 -> [w8285 _]
          tunnel: w8271 -> [_ w8324]
          tunnel: w8264 -> [_ w8322]
          tunnel: w8266 -> [_ w8325]
          tunnel: [w8283 w8303] -> w8263
          tunnel: w8265 -> [w8283 _]
          tunnel: [w8282 w8301] -> w8260
          tunnel: w8261 -> [w8282 _]
          tunnel: [w8281 w8300] -> w8257
          tunnel: w8258 -> [w8281 _]
          tunnel: "Start Saving" -> [_ w8298]
          tunnel: w8253 -> [_ w8297]
          tunnel: [w8280 w8288] -> w8246
          tunnel: w8250 -> [w8280 _]
          tunnel: [w8279 w8287] -> w8247
          tunnel: w8248 -> [w8279 _]
          frame False {
            n1830 = Increment(x=w8286) -> (x+1=w8284:i32)
          }
          frame True {
            w8294 = FALSE ("Start Saving")
            w8299 = 9.0  # File Version
            w8307 = FALSE ("prepend array or string size? (T)")
            w8305 = T31."big-endian, network order" ("byte order (0:big-endian, network order)")
            # "write file headers"
            n1831 = local read "BD 1 Frequency 1 (MHz)"() -> (w8321:dbl)
            n1832 = local read "BD 2 Frequency 1 (MHz)"() -> (w8320:dbl)
            n1833 = local read "BD 1 Frequency 2 (MHz)"() -> (w8319:dbl)
            n1834 = local read "BD 2 Frequency 2 (MHz)"() -> (w8318:dbl)
            n1835 = local read "BD 1 Frequency 3 (MHz)"() -> (w8317:dbl)
            n1836 = local read "BD 2 Frequency 3 (MHz)"() -> (w8316:dbl)
            n1837 = Array Size(array=w8297) -> (size(s)=w8296:i32)
            n1838 = To Double Precision Float(number=w8296) -> (double precision float=w8295:dbl)
            n1839 = local write "Save Calibration"(w8294) -> ()
            n1840 = local write "Start Saving"(w8294) -> ()
            n1841 = Build Array("Save APD Data\nwith Trap Data", "Save Trap Pos. Data") -> (w8291:bool[])
            n1842 = Boolean Array To Number(Boolean array=w8291) -> (number=w8290:u32)
            n1843 = Build Array(w8321, w8320, w8319, w8318, w8317, w8316) -> (w8315:dbl[])
            n1844 = case shown="4" w8325 {
              tunnel: w8324 -> [w8396 w8416 w8432 w8470]
              tunnel: w8295 -> [w8401 w8423 w8452 w8489]
              tunnel: w8322 -> [w8400 w8422 w8451 w8488]
              tunnel: [w8397 w8418 w8443 w8480] -> w8313
              tunnel: [w8388 "Cal sets to save" w8433 w8471] -> w8303
              tunnel: w8315 -> [w8398 w8419 w8445 w8482]
              tunnel: "Save APD Data\nwith Trap Data" -> [w8395 _ w8429 w8468]
              tunnel: [w8395 w8410 w8429 w8468] -> w8300
              tunnel: w8299 -> [w8391 w8411 w8427 w8466]
              tunnel: w8298 -> [w8390 _ _ _]
              tunnel: [w8381 w8410 w8426 w8456] -> w8287
              tunnel: "Save Trap Pos. Data" -> [w8381 _ w8426 w8456]
              tunnel: w8290 -> [w8380 _ w8425 w8455]
              frame 1, Default {
                # "timeseries"
                n1845 = case shown="True" "Profile" {
                  tunnel: [w8404 w8407] -> w8385
                  tunnel: [w8404 w8406] -> w8384
                  tunnel: [w8404 w8405] -> w8383
                  tunnel: [w8404 w8409] -> w8382
                  frame False {
                    w8404 = 0.0 ("f")
                  }
                  frame True {
                    n1846 = local read "Current Position"() -> (w8408:dbl[])
                    n1847 = local read "Y change (mm)"() -> (w8409:dbl)
                    n1848 = call "subVI_explode3array.vi"("Array"=w8408) -> ("x"=w8407:dbl, "y"=w8406:dbl, "z"=w8405:dbl)  [unwired: 12 in]
                  }
                }
                n1849 = local read "Save ave N"() -> (w8403:dbl)
                n1850 = Multiply(x=w8403, y=w8396) -> (x*y=w8402:dbl)
                n1851 = To Double Precision Float(number=w8380) -> (double precision float=w8394:dbl)
                n1852 = Build Array(w8391, w8396, w8402, w8401, w8400, 0.0 ("f")) -> (w8399:dbl[])
                n1853 = Build Array(w8394, w8385, w8384, w8383, w8382) -> (w8392:dbl[])
                n1854 = Select(t=u32 4000000000, s=w8390, f="N sets to save") -> (s? t:f=w8388:u32)
                n1855 = Build Array (concatenate)(w8399, w8398, w8392) -> (w8397:dbl[])
              }
              frame 2 {
                w8413 = 0.0 ("f")
                w8410 = FALSE ("Save APD Data\nwith Trap Data")
                # "calibration"
                n1856 = Boolean To (0,1)(Boolean=w8410) -> (0, 1=w8415:i16)
                n1857 = To Double Precision Float(number=w8415) -> (double precision float=w8414:dbl)
                n1858 = Build Array(w8414, w8413, w8413, w8413, w8413) -> (w8412:dbl[])
                n1859 = Build Array(w8411, w8416, w8416, w8423, w8422, 1.0 ("t")) -> (w8420:dbl[])
                n1860 = Build Array (concatenate)(w8420, w8419, w8412) -> (w8418:dbl[])
                "Calibrating Trap..." <- TRUE ("Calibrating...")
              }
              frame 4 {
                w8430 = 0.0 ("f")
                # "write file header for a trap \nraster scan"
                # "scan dir (x/y = 0/1)"
                # "cycles/step"
                # "n scans (f/b)"
                # "steps"
                # "freq. range"
                # "AOD raster scan"
                n1861 = local read "Number of F/B Scans (AOD)"() -> (w8437:u16)
                n1862 = local read "Cycles/step (AOD)"() -> (w8439:u64)
                n1863 = local read "Scan Range (MHz)"() -> (w8442:dbl)
                n1864 = local read "Scan steps (AOD)"() -> (w8441:u64)
                n1865 = local read "Scan BD"() -> (w8449:bool)
                n1866 = local read "Save ave N"() -> (w8454:dbl)
                n1867 = Boolean To (0,1)(Boolean=w8449) -> (0, 1=w8448:i16)
                n1868 = To Double Precision Float(number=w8437) -> (double precision float=w8436:dbl)
                n1869 = To Double Precision Float(number=w8441) -> (double precision float=w8440:dbl)
                n1870 = To Double Precision Float(number=w8439) -> (double precision float=w8438:dbl)
                n1871 = To Double Precision Float(number=w8448) -> (double precision float=w8447:dbl)
                n1872 = Multiply(x=w8454, y=w8432) -> (x*y=w8453:dbl)
                n1873 = To Double Precision Float(number=w8425) -> (double precision float=w8431:dbl)
                n1874 = Build Array(w8431, w8430, w8430, w8430, w8430) -> (w8428:dbl[])
                n1875 = local read "N sets should be saved"() -> (w8434:dbl)
                n1876 = Build Array(w8447, w8442, w8440, w8438, w8436) -> (w8444:dbl[])
                n1877 = Build Array(w8427, w8432, w8453, w8452, w8451, 2.0 ("t")) -> (w8446:dbl[])
                n1878 = Round Toward +Infinity(x=w8434) -> (ceil(x): smallest int >= x=w8435:dbl)
                n1879 = Build Array (concatenate)(w8446, w8445, w8428, w8444) -> (w8443:dbl[])
                n1880 = To Unsigned Long Integer(number=w8435) -> (unsigned 32bit integer=w8433:u32)
              }
              frame 8 {
                w8463 = 0.0 ("f")
                # "MCL raster scan"
                n1881 = local read "Number of scans (MCL)"() -> (w8458:u64)
                n1882 = local read "Scan lines (y)"() -> (w8457:u64)
                n1883 = local read "2D or 1D Scan"() -> (w8460:bool)
                n1884 = local read "Scan Range (V)\n(of steps)"() -> (w8479:dbl)
                n1885 = local read "Fast Scan Dir"() -> (w8486:bool)
                n1886 = local read "Cycles/step (MCL)"() -> (w8476:u64)
                n1887 = local read "Scan steps (MCL)"() -> (w8478:u64)
                n1888 = Select(t=w8457, s=w8460, f=w8458) -> (s? t:f=w8459:u64)
                n1889 = Boolean To (0,1)(Boolean=w8460) -> (0, 1=w8462:i16)
                n1890 = local read "Save ave N"() -> (w8491:dbl)
                n1891 = local read "Initial X"() -> (w8465:dbl)
                n1892 = local read "Initial Y"() -> (w8464:dbl)
                n1893 = To Double Precision Float(number=w8462) -> (double precision float=w8461:dbl)
                n1894 = Boolean To (0,1)(Boolean=w8486) -> (0, 1=w8485:i16)
                n1895 = To Double Precision Float(number=w8459) -> (double precision float=w8474:dbl)
                n1896 = To Double Precision Float(number=w8478) -> (double precision float=w8477:dbl)
                n1897 = To Double Precision Float(number=w8476) -> (double precision float=w8475:dbl)
                n1898 = To Double Precision Float(number=w8485) -> (double precision float=w8484:dbl)
                n1899 = Multiply(x=w8491, y=w8470) -> (x*y=w8490:dbl)
                n1900 = To Double Precision Float(number=w8455) -> (double precision float=w8469:dbl)
                n1901 = local read "N sets should be saved (MCL)"() -> (w8472:dbl)
                n1902 = Build Array(w8469, w8461, w8463, w8463, w8463) -> (w8467:dbl[])
                n1903 = Build Array(w8484, w8479, w8477, w8475, w8474, w8465, w8464) -> (w8481:dbl[])
                n1904 = Build Array(w8466, w8470, w8490, w8489, w8488, 3.0 ("t")) -> (w8483:dbl[])
                n1905 = Round Toward +Infinity(x=w8472) -> (ceil(x): smallest int >= x=w8473:dbl)
                n1906 = Build Array (concatenate)(w8483, w8482, w8467, w8481) -> (w8480:dbl[])
                n1907 = To Unsigned Long Integer(number=w8473) -> (unsigned 32bit integer=w8471:u32)
              }
            }
            n1908 = local read "Index"() -> (w8330:dbl)
            n1909 = call "Create new save file.vi"("Insert"="", "Ext"=".dat", "Index In"=w8330) -> ("Path Out"=w8289:path, "Index Out"=w8302:dbl)
            n1910 = local write "Save file name"(w8289) -> ()
            n1911 = local write "Index"(w8302) -> ()
            n1912 = local write "Save index"(w8302) -> ()
            n1913 = Array Size(array=w8313) -> (size(s)=w8314:i32)
            n1914 = Open/Create/Replace File(file path (use dialog)=w8289, operation (0:open)=T25."create", access (0:read/write)=enum16{"read/write", "read-only", "write-only"}."write-only") -> (refnum out=w8327:refnum<file>)  [unwired: 1 in, 4 out]
            n1915 = local write "Saving..."(TRUE ("Saving...")) -> ()
            n1916 = To Double Precision Float(number=w8314) -> (double precision float=w8312:dbl)
            n1917 = String Length(string="Comment (data description)") -> (length=w8310:i32)
            n1918 = To Double Precision Float(number=w8310) -> (double precision float=w8309:dbl)
            n1919 = Deny Access(7:w8327) -> (3:w8326:refnum<file>)  [unwired: 1 in, 2 out]
            n1920 = Build Array (concatenate)(w8312, w8313, w8309) -> (w8311:dbl[])
            n1921 = case "If fluorescence data to be saved" shown="True" w8300 {
              tunnel: w8289 -> [_ w8379]
              tunnel: [refnum<k0> refnum w8359] -> w8301
              frame False {
              }
              frame True {
                w8358 = 0.0
                n1922 = local read "APD Integration Time (s)"() -> (w8364:dbl)
                n1923 = local read "N APD Samp/step"() -> (w8357:dbl)
                n1924 = Path To String(path=w8379) -> (string=w8378:string)
                n1925 = String Length(string=w8378) -> (length=w8377:i32)
                n1926 = Subtract(x=w8377, y=4) -> (x-y=w8375:i32)
                n1927 = String Subset(string=w8378, length (rest)=w8375) -> (substring=w8374:string)  [unwired: 1 out]
                n1928 = Build Array(w8364, w8357, w8358, w8358, w8358, w8358, w8358, w8358) -> (w8361:dbl[])
                n1929 = Concatenate Strings(w8374, "_fl.dat" ("string")) -> (w8372:string)
                n1930 = Array Size(array=w8361) -> (size(s)=w8363:i32)
                n1931 = String To Path(string=w8372) -> (path=w8368:path)
                n1932 = Open/Create/Replace File(file path (use dialog)=w8368, operation (0:open)=T25."create", access (0:read/write)=enum16{"read/write", "read-only", "write-only"}."write-only") -> (refnum out=w8369:refnum<file>)  [unwired: 1 in, 4 out]
                n1933 = Deny Access(7:w8369) -> (3:w8365:refnum<file>)  [unwired: 1 in, 2 out]
                n1934 = To Double Precision Float(number=w8363) -> (double precision float=w8362:dbl)
                n1935 = Build Array (concatenate)(w8362, w8361) -> (w8360:dbl[])
                n1936 = Write to Binary File(file (use dialog)=w8365, data=w8360, 5:FALSE ("prepend array or string size? (T)"), 9:T31."big-endian, network order" ("byte order (0:big-endian, network order)")) -> (refnum out=w8359:refnum<file>)  [unwired: 1 in, 3 out]
              }
            }
            n1937 = case shown="True" w8287 {
              tunnel: w8289 -> [_ w8341]
              tunnel: [refnum<k0> refnum w8340] -> w8288
              frame False {
              }
              frame True {
                w8336 = 0.0 ("element")
                n1938 = Path To String(path=w8341) -> (string=w8355:string)
                n1939 = Build Array(w8336, w8336, w8336, w8336, w8336, w8336, w8336, w8336) -> (w8337:dbl[])
                n1940 = String Length(string=w8355) -> (length=w8354:i32)
                n1941 = Subtract(x=w8354, y=4) -> (x-y=w8352:i32)
                n1942 = Array Size(array=w8337) -> (size(s)=w8339:i32)
                n1943 = String Subset(string=w8355, length (rest)=w8352) -> (substring=w8351:string)  [unwired: 1 out]
                n1944 = To Double Precision Float(number=w8339) -> (double precision float=w8338:dbl)
                n1945 = Concatenate Strings(w8351, "_pos.dat" ("string")) -> (w8349:string)
                n1946 = Build Array (concatenate)(w8338, w8337) -> (w8335:dbl[])
                n1947 = String To Path(string=w8349) -> (path=w8345:path)
                n1948 = Open/Create/Replace File(file path (use dialog)=w8345, operation (0:open)=T25."create", access (0:read/write)=enum16{"read/write", "read-only", "write-only"}."write-only") -> (refnum out=w8346:refnum<file>)  [unwired: 1 in, 4 out]
                n1949 = Deny Access(7:w8346) -> (3:w8342:refnum<file>)  [unwired: 1 in, 2 out]
                n1950 = Write to Binary File(file (use dialog)=w8342, data=w8335, 5:FALSE ("prepend array or string size? (T)"), 9:T31."big-endian, network order" ("byte order (0:big-endian, network order)")) -> (refnum out=w8340:refnum<file>)  [unwired: 1 in, 3 out]
              }
            }
            n1951 = Write to Binary File(file (use dialog)=w8326, data=w8311, 5:w8307, 9:w8305) -> (refnum out=w8308:refnum<file>)  [unwired: 1 in, 3 out]
            n1952 = Write to Binary File(file (use dialog)=w8308, data="Comment (data description)", 5:w8307, 9:w8305) -> (refnum out=w8304:refnum<file>)  [unwired: 1 in, 3 out]
          }
        }
        n1953 = feedback-in #19(w8247) -> ()
        n1954 = feedback-in #20(w8274) -> ()
        n1955 = feedback-in #21(w8246) -> ()
        n1956 = feedback-in #22(w8257) -> ()
        n1957 = feedback-in #23(w8260) -> ()
        n1958 = feedback-in #24(w8273) -> ()
        n1959 = feedback-in #25(w8263) -> ()
      }
      frame #1 {
        n1960 = local read "Saving..."() -> (w8504:bool)
        n1961 = case shown="True" w8504 {
          tunnel: w8508 -> [_ w8518]
          tunnel: w8507 -> [_ w8532]
          tunnel: w8506 -> [_ w8528]
          tunnel: w8505 -> [_ w8527]
          tunnel: w8503 -> [_ w8526]
          tunnel: w8502 -> [_ w8521]
          tunnel: w8501 -> [_ w8520]
          tunnel: w8500 -> [_ w8519]
          tunnel: w8499 -> [_ w8517]
          tunnel: w8498 -> [_ w8515]
          tunnel: w8497 -> [_ w8514]
          tunnel: w8496 -> [_ w8513]
          tunnel: w8495 -> [_ w8512]
          tunnel: w8494 -> [_ w8511]
          tunnel: w8493 -> [_ w8510]
          tunnel: w8492 -> [_ w8509]
          frame False {
          }
          frame True {
            n1962 = Multiply(x=w8518, y=w8517) -> (x*y=→"Time (s)":dbl)
            n1963 = Less Or Equal?(x=w8518, y=w8526) -> (x <= y?=w8530:bool)
            n1964 = Or(x="Stop Saving", y="Abort save 2") -> (x .or. y?=w8522:bool)
            n1965 = Not(x=w8522) -> (.not. x?=w8531:bool)
            n1966 = And(x=w8530, y=w8531) -> (x .and. y?=w8529:bool)
            n1967 = case shown="False" w8529 {
              tunnel: w8532 -> [w8539 w8607]
              tunnel: [0.0 w8610] -> w8525
              tunnel: w8518 -> [_ w8608]
              tunnel: w8526 -> [_ w8609]
              tunnel: w8528 -> [_ w8604]
              tunnel: w8527 -> [_ _]
              tunnel: w8521 -> [w8537 w8597]
              tunnel: w8520 -> [w8536 w8598]
              tunnel: w8519 -> [_ w8596]
              tunnel: w8515 -> [_ w8595]
              tunnel: w8514 -> [_ w8549]
              tunnel: w8513 -> [_ w8588]
              tunnel: w8512 -> [_ w8566]
              tunnel: w8511 -> [w8534 w8547]
              tunnel: w8510 -> [w8535 w8546]
              tunnel: w8509 -> [_ w8543]
              frame False {
                w8533 = FALSE
                n1968 = Close File(refnum=w8539) -> ()  [unwired: 1 in, 2 out]
                n1969 = case shown="True" w8536 {
                  tunnel: w8537 -> [_ w8541]